vi "HFRR ADV v040.vi"() -> ()   [LabVIEW 2025] (continued)
            w2089 = u32 10000  # timeout (10sec)
            n1729 = VISA Close(VISA resource name=w2084, error in (no error)=w2082) -> (error out=w2085:errorcluster)
            n1730 = local write "Port 1a"(FALSE ("Port 1a")) -> ()
            n1731 = local read "Com Port 1"() -> (w2079:refnum<visa-resource-name>)
            n1732 = call <vilib>:"Clear Errors.vi"("error in (no error)"=w2085) -> ("error out"=w2083:errorcluster)  [unwired: 5 in, 1 out]
            n1733 = call-poly "VISA Configure Serial Port"("VISA resource name"=w2079, "timeout (10sec)"=w2089, "baud rate (9600)"=u32 250000 ("baud rate  2"), "data bits (8)"=u16 8 ("data bits  2"), "parity (0:none)"=w2088, "error in (no error)"=w2083, "stop bits (10: 1 bit)"=w2090, "flow control (0:none)"=w2092) -> ("VISA resource name out"=w2093:refnum<visa-resource-name>, "error out"=w2094:errorcluster)  [unwired: 6 in]
            n1734 = flat-sequence {
              tunnel: w2093 -> [w2096]
              tunnel: w2094 -> [w2095]
              tunnel: [w2096] -> w2086
              tunnel: [w2095] -> w2080
              frame #0 {
                n1735 = Wait (ms)(milliseconds to wait=u32 50) -> ()  [unwired: 1 out]
              }
            }
            "Residual Uno" <- ""
          }
        }
        n1736 = local read "Quit"() -> (w2041:bool)
        "Error Uno" <- w2046
      }
      n1737 = VISA Close(VISA resource name=w2039, error in (no error)=w2038) -> (error out=w2036:errorcluster)
      n1738 = call <vilib>:"Clear Errors.vi"("error in (no error)"=w2036) -> ()  [unwired: 5 in, 2 out]
    }
    frame Enabled {
    }
  }
  n1739 = while {
    stop <- w2107 stop-if-true
    # "V0OLTAGE TO STROKE (peice vise calibration)"
    n1740 = local read "LVDT MIN"() -> (w2099:dbl)
    n1741 = local read "LVDT Peak"() -> (w2098:dbl)
    n1742 = Wait (ms)(milliseconds to wait=u32 10) -> ()  [unwired: 1 out]
    n1743 = formula code="// Dynamic Parameterized Linear Interpolation Node\n// Inputs: vpp_val, voltages (Array), distances (Array)\n// Outputs: stroke\n\nint i = 0;\nint segments = 11; // 12 points make 11 interpolation segments\n\n// 1. Lower Boundary Clamp\nif (vpp_val <= voltages[0]) {\n    stroke = distances[0];\n}\n// 2. Upper Boundary Clamp\nelse if (vpp_val >= voltages[segments]) {\n    stroke = distances[segments];\n}\n// 3. Dynamic Segment Search Loop\nelse {\n    stroke = distances[0]; // Fallback baseline\n    for (i = 0; i < segments; i++) {\n        if (vpp_val >= voltages[i] && vpp_val <= voltages[i+1]) {\n            // Standard linear interpolation formula using array lookups\n            stroke = distances[i] + (vpp_val - voltages[i]) * (distances[i+1] - distances[i]) / (voltages[i+1] - voltages[i]);\n            break; // Segment found, safely exit the loop\n        }\n    }\n}"("vpp_val"=w2098, "voltages"="calibration values", "distances"="STROKE") -> ("stroke"=→"LVDT STROKE":dbl)
    n1744 = local read "Calibration Tare Value"() -> (w2103:dbl)
    n1745 = local read "Calibration Tare"() -> (w2101:bool)
    n1746 = Subtract(x=w2099, y=w2103) -> (x-y=→"LVDT STROKE  Calibration":dbl)
    n1747 = case shown="True" w2101 {
      selector: w2101 -> [_ w2109]
      tunnel: w2099 -> [_ w2110]
      frame False {
      }
      frame True {
        n1748 = Not(x=w2109) -> (.not. x?=w2108:bool)
        n1749 = local write "Calibration Tare"(w2108) -> ()
        "Calibration Tare Value" <- w2110
      }
    }
    n1750 = local read "Quit"() -> (w2107:bool)
  }
  n1751 = while {
    stop <- w2133 stop-if-true
    n1752 = local read "Due read"() -> (w2131:string)
    n1753 = call <vilib>:"High Resolution Polling Wait.vi"("seconds to wait"=0.02) -> ()  [unwired: 10 in, 1 out]
    n1754 = local read "Frictioin Force Raw"() -> (w2113:dbl)
    n1755 = Spreadsheet String To Array(delimiter (Tab)=";", format string="", spreadsheet string=w2131, array type (2D Dbl)=string[] []) -> (array=w2128:string[])
    n1756 = Fract/Exp String To Number(string=w2128) -> (number=w2127:dbl[])  [unwired: 3 in, 1 out]
    n1757 = call <vilib>:"Median Filter PtByPt.vi"("rank"=2, "x"=w2113) -> ("Filtered x"=→"Friction":dbl)  [unwired: 2 in, 1 out]
    n1758 = Index Array(array=w2127) -> (element #1=→"Sample Temperature":dbl, element #2=→"Target Sample Temperature":dbl, element #3=→"Current Duty Cycle":dbl, element #4=→"Ambient Temperature":dbl, element #5=→"Dac Status":dbl, element #6=→"Vpp":dbl, element #7=→"Active Error Code":dbl, element #8=→"Kp":dbl, element #9=→"Ki":dbl, element #10=→"Kd":dbl, element #11=→"SampleRaw":dbl, element #12=→"AmbRaw":dbl)  [unwired: 12 in]
    n1759 = local read "Quit"() -> (w2133:bool)
  }
  n1760 = while {
    shift-right: [w2147] -> w43
    shift-left: _ -> [w2139]
    shift-right: [w2134] -> w42
    shift-left: errorcluster {"status"=FALSE, "code"=0, "source"="Init"} ("error out") -> [w2141]
    tunnel: [w2136] -> w46
    tunnel: [w2146] -> _
    i -> [w2146]
    stop <- w2136 stop-if-true
    n1761 = local read "Com Port 2"() -> (w2140:refnum<visa-resource-name>)
    n1762 = local read "Port 2a"() -> (w2142:bool)
    n1763 = Unbundle(w2141) -> ("status"=→"Port 4":bool)  [unwired: 2 out]
    n1764 = call <vilib>:"High Resolution Polling Wait.vi"("seconds to wait"=0.02) -> ()  [unwired: 10 in, 1 out]
    n1765 = local read "Port 4"() -> (w2143:bool)
    n1766 = Not Equal?(x=w2140, y=w2139) -> (x != y?=w2138:bool)
    n1767 = Or(x=w2143, y=w2142) -> (x .or. y?=w2145:bool)
    n1768 = case shown="False" w2145 {
      frame False {
        w2150 = TRUE ("Visible")
        n1769 = property on="Port 2a" class="Bool (strict)"("Visible"=w2150) -> ()  [unwired: 2 in, 2 out]
        n1770 = property on="Port 4" class="Bool (strict)"("Visible"=w2150) -> ()  [unwired: 2 in, 2 out]
      }
      frame True {
        w2151 = TRUE ("Visible")
        n1771 = property on="Port 2a" class="Bool (strict)"("Visible"=w2151) -> ()  [unwired: 2 in, 2 out]
        n1772 = property on="Port 4" class="Bool (strict)"("Visible"=w2151) -> ()  [unwired: 2 in, 2 out]
      }
    }
    n1773 = case shown="True" w2138 {
      tunnel: [w2148 errorcluster {"status"=TRUE, "code"=0, "source"="Init"} ("error out")] -> w2137
      tunnel: w2141 -> [w2148 _]
      frame False {
      }
      frame True {
      }
    }
    n1774 = case shown="No Error" w2137 {
      selector: w2137 -> [w2164 w2195]
      tunnel: [w2157 w2200] -> w2147
      tunnel: [w2165 w2193] -> w2134
      tunnel: w2139 -> [w2166 w2198]
      frame No Error {
        n1775 = property class="Instr" props=["Serial Settings:Number of Bytes at Serial Port"](reference=w2166, error in=w2164) -> (reference out=w2158:refnum<visa-resource-name>, error out=w2163:errorcluster)  [unwired: 1 out]
        n1776 = while {
          tunnel: [w2174] -> w2159
          tunnel: [w2173] -> w2160
          tunnel: w2163 -> [w2172]
          tunnel: w2158 -> [w2171]
          tunnel: [w2170] -> _
          i -> [w2170]
          stop <- TRUE stop-if-true
          n1777 = property class="Instr" props=["Serial Settings:Number of Bytes at Serial Port"](reference=w2171, error in=w2172) -> (reference out=w2176:refnum<visa-resource-name>, error out=w2175:errorcluster)  [unwired: 1 out]
          n1778 = VISA Read(VISA resource name=w2176, byte count=u32 1000, error in (no error)=w2175) -> (VISA resource name out=w2173:refnum<visa-resource-name>, read buffer=→"Due read":string, error out=w2174:errorcluster)  [unwired: 1 out]
        }
        n1779 = local read "Due Write"() -> (w2156:string)
        n1780 = call <vilib>:"Trim Whitespace.vi"("string"=w2156) -> ("trimmed string"=w2155:string)  [unwired: 1 in]
        n1781 = Not Equal?(x=w2155, y="") -> (x != y?=w2161:bool)
        n1782 = VISA Flush I/O Buffer(VISA resource name=w2160) -> (VISA resource name out=w2153:refnum<visa-resource-name>, error out=→"error out 10":errorcluster)  [unwired: 2 in]
        n1783 = case shown="True" w2161 {
          tunnel: w2153 -> [w2178 w2183]
          tunnel: [w2178 w2187] -> w2157
          tunnel: w2159 -> [w2177 w2182]
          tunnel: [w2177 w2185] -> w2165
          tunnel: w2155 -> [_ w2181]
          tunnel: [_ w2184] -> _
          frame False {
            # "DATA  WRITE LOOP"
          }
          frame True {
            n1784 = Concatenate Strings(w2181, "\r\n") -> (w2180:string)
            n1785 = VISA Write(VISA resource name=w2183, write buffer=w2180, error in (no error)=w2182) -> (VISA resource name out=w2187:refnum<visa-resource-name>, return count=w2184:u32, error out=w2186:errorcluster)
            n1786 = flat-sequence {
              tunnel: w2186 -> [w2189]
              tunnel: [w2189] -> w2185
              frame #0 {
                n1787 = local write "Due Write"("" ("Command")) -> ()
                n1788 = Wait (ms)(milliseconds to wait=u32 5) -> ()  [unwired: 1 out]
              }
            }
          }
        }
        "Port 2a" <- TRUE ("Port 2a")
      }
      frame Error {
        w2206 = u16 0 items=["None", "XON/XOFF", "RTS/CTS", "XON/XOFF & RTS/CTS", "DTR/DSR", "XON/XOFF & DTR/DSR"] ("flow control (0:none)  2")
        w2204 = u16 10 items=["1.0"=10, "1.5"=15, "2.0"=20] ("stop bits 2")
        w2202 = u16 0 items=["None", "Odd", "Even", "Mark", "Space"] ("parity 2")
        w2203 = u32 10000  # timeout (10sec)
        n1789 = VISA Clear(VISA resource name=w2198, error in (no error)=w2195) -> (VISA resource name out=w2197:refnum<visa-resource-name>, error out=w2196:errorcluster)
        n1790 = VISA Close(VISA resource name=w2197, error in (no error)=w2196) -> (error out=w2199:errorcluster)
        n1791 = call <vilib>:"Clear Errors.vi"("error in (no error)"=w2199) -> ()  [unwired: 5 in, 2 out]
        n1792 = local write "Port 2a"(FALSE ("Port 2a")) -> ()
        n1793 = local read "Com Port 2"() -> (w2192:refnum<visa-resource-name>)
        "visa due" <- w2192
        n1794 = call-poly "VISA Configure Serial Port"("VISA resource name"=w2192, "timeout (10sec)"=w2203, "baud rate (9600)"=u32 250000 ("baud rate  2"), "data bits (8)"=u16 8 ("data bits  2"), "parity (0:none)"=w2202, "stop bits (10: 1 bit)"=w2204, "flow control (0:none)"=w2206) -> ("VISA resource name out"=w2207:refnum<visa-resource-name>, "error out"=w2208:errorcluster)  [unwired: 7 in]
        n1795 = flat-sequence {
          tunnel: w2207 -> [w2210]
          tunnel: w2208 -> [w2209]
          tunnel: [w2210] -> w2200
          tunnel: [w2209] -> w2193
          frame #0 {
            n1796 = Wait (ms)(milliseconds to wait=u32 50) -> ()  [unwired: 1 out]
          }
        }
        "Residual Due" <- ""
      }
    }
    "error out 9" <- w2134
    n1797 = local read "Quit"() -> (w2136:bool)
    "Error Due" <- w2141
  }
  n1798 = local write "FRICVALZ"(0.0 ("FRICVALZ")) -> ()
  n1799 = property on="RUN" class="Bool (strict)"("Visible"=TRUE) -> ()  [unwired: 2 in, 2 out]
  n1800 = while {
    tunnel: [w2225] -> _
    tunnel: [w2212] -> w56
    i -> [w2225]
    stop <- w2212 stop-if-true
    n1801 = local read "conststatus"() -> (w2216:dbl)
    n1802 = local read "Main Tab"() -> (w2214:T2)
    n1803 = local read "EDIT"() -> (w2231:bool)
    n1804 = local read "Rate"() -> (w2230:dbl)
    n1805 = case shown="True" w2231 {
      tunnel: [FALSE TRUE] -> _
      frame False {
      }
      frame True {
      }
    }
    n1806 = Equal?(x=w2214, y=T29."About" ("Main Tab")) -> (x = y?=w2223:bool)
    n1807 = Equal?(x=w2216, y=0.0) -> (x = y?=w2217:bool)
    n1808 = Divide(x=1.0, y=w2230) -> (x/y=w2226:dbl)
    "Time 2" <- w2226
    n1809 = case shown="True" w2217 {
      frame False {
      }
      frame True {
        # "C:\\WinDucom\\calibrate WO 2391.dcf"
        n1810 = local write "Lan flag"(22) -> ()
        n1811 = local write "conststatus"(10.0 ("rpm value : 2")) -> ()
        n1812 = String To Path(string="C:\\LAB-IQ\\calibrate WO 2465.dcf") -> (path=w2237:path)
        n1813 = Open/Create/Replace File "Open File"(file path (use dialog)=w2237) -> (refnum out=w2235:refnum<file>)  [unwired: 5 in, 2 out]
        n1814 = for {
          N: 23 -> [_]
          tunnel: w2235 -> [w2246]
          i -> [w2240]
          (unwired) TRUE ("line mode (F)")
          n1815 = Read from Text File "Read File"(file (use dialog)=w2246) -> (text=w2245:string)  [unwired: 3 in, 3 out]
          n1816 = Match Pattern(string=w2245, regular expression="]") -> (after substring=w2243:string)  [unwired: 1 in, 3 out]
          n1817 = String Subset(string=w2245, offset (0)=5, length (rest)=10 ("length (rest)")) -> (substring=w2238:string)
          n1818 = Fract/Exp String To Number(string=w2238) -> (number=w2239:dbl)  [unwired: 3 in, 1 out]
          n1819 = Match Pattern(string=w2243, regular expression="-") -> (before substring=w2241:string)  [unwired: 1 in, 3 out]
          n1820 = case shown="10" w2240 {
            tunnel: w2239 -> [_ _ _ _ _ _ _ _ _ _ w2253 _ _ _ _ _ _ _ _ _ _ _ _ _]
            tunnel: w2241 -> [_ _ _ _ w2249 w2250 w2251 _ _ _ _ _ _ _ _ _ _ _ _ _ w2254 w2255 w2256 _]
            frame 0 {
            }
            frame 1 {
            }
            frame 2 {
            }
            frame 3 {
            }
            frame 4 {
              n1821 = local write "Com Port 1"(w2249) -> ()
            }
            frame 5 {
              n1822 = local write "Com Port 2"(w2250) -> ()
              n1823 = local write "visa due"(w2250) -> ()
            }
            frame 6 {
              n1824 = String To Path(string=w2251) -> (path=w2252:path)
              n1825 = local write "File Path"(w2252) -> ()
              "String" <- w2251
            }
            frame 7 {
            }
            frame 8 {
            }
            frame 9 {
            }
            frame 10 {
              n1826 = local write "Language Selection"(w2253) -> ()
            }
            frame 11 {
            }
            frame 12 {
            }
            frame 13 {
            }
            frame 14 {
            }
            frame 15 {
            }
            frame 16 {
            }
            frame 17 {
            }
            frame 18 {
            }
            frame 21 {
            }
            frame 22 {
              n1827 = local write "Com Port 3"(w2254) -> ()
            }
            frame 20 {
              n1828 = local write "Camera Port :"(w2255) -> ()
            }
            frame 19 {
              n1829 = local write "C3 :"(w2256) -> ()
            }
            frame 23, Default {
            }
          }
        }
      }
    }
    n1830 = Select(t=u32 2500 ("milliseconds to wait"), s=w2223, f=u32 500 ("milliseconds to wait")) -> (s? t:f=w2221:u32)
    n1831 = Multiply(x=w2226, y=w2221) -> (x*y=w2228:dbl)
    n1832 = call "Elapsed Time2"("Time Target (s)"=w2228, "Auto Reset"=TRUE) -> ("Time has Elapsed"=w2218:bool)  [unwired: 10 in, 7 out]
    n1833 = case shown="True" w2218 {
      frame False {
      }
      frame True {
        n1834 = stacked-sequence {
          frame #0 {
            # "DATA PROCESSING"
            # "115 mV/N"
            n1835 = local read "Sample Temperature"() -> (w2259:dbl)
            n1836 = local read "RH Numeric:"() -> (→"Humidity ( %RH )":dbl)
            n1837 = local read "FRICVALZ"() -> (w2276:dbl)
            n1838 = local read "Friction"() -> (w2262:dbl)
            n1839 = call <vilib>:"Mean PtByPt.vi"("x"=w2259, "sample length"=100) -> ("mean"=w2258:dbl)  [unwired: 2 in, 1 out]
            "TEMP 2" <- w2258
            "TEMP 3" <- w2258
            n1840 = Subtract(x=w2262, y=w2276) -> (x-y=w2271:dbl)
            "FF 2" <- w2271
            "FF 4" <- w2271
            n1841 = local read "Ambient Temperature"() -> (→"AIR TEMP":dbl)
            n1842 = local read "TEMP"() -> (w2275:dbl)
            n1843 = local write "FF 3"(w2271) -> ()
            n1844 = Compound Arithmetic op=OR("FRICVALZ 4", "FRICVALZ 3", "FRICVALZ 2") -> (w2267:bool)
            n1845 = case shown="True" w2267 {
              tunnel: w2262 -> [_ w2282]
              frame False {
              }
              frame True {
                w2281 = FALSE ("FRICVALZ")
                n1846 = local write "FRICVALZ 3"(w2281) -> ()
                n1847 = local write "FRICVALZ 2"(w2281) -> ()
                n1848 = local write "FRICVALZ 4"(w2281) -> ()
                "FRICVALZ" <- w2282
              }
            }
            n1849 = Not A Number/Path/Refnum?(number/path/refnum=w2275) -> (NaN/Path/Refnum?=w2274:bool)
            n1850 = Not A Number/Path/Refnum?(number/path/refnum=w2271) -> (NaN/Path/Refnum?=w2273:bool)
            n1851 = Divide(x=w2271, y=1.96) -> (x/y=w2268:dbl)
            n1852 = Compound Arithmetic op=OR(w2274, w2273) -> (w2272:bool)
            n1853 = Not A Number/Path/Refnum?(number/path/refnum=w2268) -> (NaN/Path/Refnum?=w2269:bool)
            n1854 = case shown="True" w2272 {
              frame False {
              }
              frame True {
                n1855 = local write "TEMP"(0.0 ("TEMP")) -> ()
                n1856 = local write "FF 2"(0.0 ("FF 2")) -> ()
                n1857 = local write "reinit"(TRUE ("reinit")) -> ()
              }
            }
            n1858 = local write "TEMP"(w2258) -> ()
            n1859 = Select(t=0.0, s=w2269, f=w2268) -> (s? t:f=w2261:dbl)
            "COF 2" <- w2261
            n1860 = local write "COF 3"(w2261) -> ()
          }
        }
      }
    }
    n1861 = Wait (ms)(milliseconds to wait=u32 50) -> ()  [unwired: 1 out]
    n1862 = local read "Quit"() -> (w2212:bool)
    "Rate" <- 2500.0 ("No of Samples")
  }
  n1863 = while {
    tunnel: [w2302] -> _
    tunnel: [w2285] -> w58
    tunnel: w3 -> [_]
    i -> [w2302]
    stop <- w2285 stop-if-true
    # "C:\\LAB-IQ-NXT\\Scar View.exe"
    n1864 = local read "OK Button 16"() -> (w2292:bool)
    n1865 = local read "Main Tab"() -> (w2286:T2)
    n1866 = local read "service 3"() -> (w2287:bool)
    n1867 = local read "OPEN 6"() -> (w2289:bool)
    n1868 = local read "EDIT 2"() -> (w2291:bool)
    n1869 = flat-sequence {
      frame #0 {
        n1870 = stacked-sequence {
          frame #0 {
            n1871 = local read "EDIT"() -> (w2780:bool)
            n1872 = case shown="False" w2780 {
              tunnel: [u8 2 ("Disabled") u8 0 ("Disabled")] -> _
              frame False {
                w2782 = FALSE
                n1873 = local write "Password"("") -> ()
                n1874 = local write "x = y?"(w2782) -> ()
                n1875 = property on="Password" class="Str"("Visible"=w2782) -> ()  [unwired: 2 in, 2 out]
              }
              frame True {
                n1876 = property on="Password" class="Str"("Visible"=TRUE) -> ()  [unwired: 2 in, 2 out]
              }
            }
            "dipl pwd" <- "@143$\n" ("dipl pwd")
          }
          frame #1 {
          }
          frame #2 {
          }
          frame #3 {
          }
          frame #4 {
            n1877 = String To Byte Array(string="Password") -> (unsigned byte array=w2793:u8[])
            n1878 = Search 1D Array(1D array=w2793, element=u8 10) -> (index of element=w2791:i32)  [unwired: 1 in]
            n1879 = Index Array(array=w2793, index=w2791) -> (element=w2792:u8)
            n1880 = Equal?(x=w2792, y=10) -> (x = y?=w2788:bool)
            n1881 = case shown="True" w2788 {
              frame False {
              }
              frame True {
                # "password"
                # "password"
                n1882 = local read "Password"() -> (w2805:string)
                n1883 = String To Byte Array(string=w2805) -> (unsigned byte array=w2808:u8[])
                n1884 = String To Byte Array(string="@143$\n") -> (unsigned byte array=w2795:u8[])
                n1885 = Array Size(array=w2808) -> (size(s)=w2804:i32)
                n1886 = Array Size(array=w2795) -> (size(s)=w2800:i32)
                n1887 = for {
                  N: w2804 -> [_]
                  tunnel: w2808 -> [w2821]
                  tunnel: [w2819] -> w2809 mode=indexing
                  tunnel: w2804 -> [w2816]
                  i -> [w2817]
                  n1888 = Decrement(x=w2816) -> (x-1=w2815:i32)
                  n1889 = Index Array(array=w2821, index=w2817) -> (element=w2820:u8)
                  n1890 = Equal?(x=w2817, y=w2815) -> (x = y?=w2814:bool)
                  n1891 = Number To Decimal String(number=w2820) -> (decimal integer string=w2818:string)  [unwired: 1 in]
                  n1892 = Select(t="", s=w2814, f="\r") -> (s? t:f=w2811:string)
                  n1893 = Concatenate Strings(w2818, w2811) -> (w2819:string)
                }
                n1894 = for {
                  N: w2800 -> [_]
                  tunnel: w2795 -> [w2832]
                  tunnel: [w2830] -> w2798 mode=indexing
                  tunnel: w2800 -> [w2827]
                  i -> [w2828]
                  n1895 = Decrement(x=w2827) -> (x-1=w2826:i32)
                  n1896 = Index Array(array=w2832, index=w2828) -> (element=w2831:u8)
                  n1897 = Equal?(x=w2828, y=w2826) -> (x = y?=w2825:bool)
                  n1898 = Number To Decimal String(number=w2831) -> (decimal integer string=w2829:string)  [unwired: 1 in]
                  n1899 = Select(t="", s=w2825, f="\r") -> (s? t:f=w2822:string)
                  n1900 = Concatenate Strings(w2829, w2822) -> (w2830:string)
                }
                n1901 = local read "file path"() -> (w2794:path)
                n1902 = call <vilib>:"Read Characters From File.vi"("file path (dialog if empty)"=w2794) -> ("character string"=w2807:string)  [unwired: 5 in, 3 out]
                "string" <- w2807
                n1903 = flat-sequence {
                  tunnel: [w2810] -> _
                  frame #0 {
                    w2810 = ""
                    n1904 = local write "Password"(w2810) -> ()
                  }
                }
                n1905 = Concatenate Strings(w2798) -> (w2799:string)
                n1906 = Concatenate Strings(w2807) -> (w2806:string)
                n1907 = Concatenate Strings(w2809) -> (w2802:string)
                n1908 = Equal?(x=w2802, y=w2806) -> (x = y?=w2797:bool)
                n1909 = Equal?(x=w2802, y=w2799) -> (x = y?=w2803:bool)
                n1910 = Or(x=w2797, y=w2803) -> (x .or. y?=→"x = y?":bool)
              }
            }
          }
        }
        n1911 = local read "x = y?"() -> (w2778:bool)
        n1912 = And(x="EDIT", y=w2778) -> (x .and. y?=w2776:bool)
        n1913 = case shown="True" w2776 {
          tunnel: [u8 2 ("Disabled") u8 0 ("Disabled")] -> w2775
          tunnel: [w2982 TRUE ("Visible")] -> w2774
          frame False {
            w2982 = FALSE ("Visible")
            n1914 = local write "EDIT 2"(w2982) -> ()
          }
          frame True {
          }
        }
        n1915 = case shown="True" "SAVE" {
          frame False {
          }
          frame True {
            n1916 = stacked-sequence {
              seq-local: [w2837 _ _] -> [_ w2978 _]
              frame #0 {
                w2833 = 0.0 ("number")
                w2834 = 0.0 ("number")
                (unwired) i16 5 ("precision (6)")
                # "[CH1]    - FF\n[CH2]   - TEMPERATURE\n[CH3]    - Humidity\n[CH4]    - AIR TEMP\n[CH5]\\- Visa Uno\n[CH6] \\- Visa Due\n[CH7]  \\- file path\n[CH8]   - Displacement Gain\n[CHA]   - Stroke Gain\n[CHB]   - Stroke PID Gain\n[CHC]   -Language Selection\n[CHD]   -Power +\n[CHE]   -Power_\n[CHF]   -Heater\n[CHG]   -Humidity Wet\n[CHH]   -Humidity Dry\n[CHI]   -Integral Time"
                n1917 = local read "Language Selection"() -> (w2880:enum16{"English", "Russian"})
                n1918 = Path To String(path="File Path") -> (string=w2896:string)
                n1919 = Number To Fractional String(number=w2833, width (-)=i16 10 ("precision (6)"), precision (6)=i16 5) -> (F-format string=w2887:string)  [unwired: 1 in]
                n1920 = Number To Fractional String(number=w2880, width (-)=i16 10 ("precision (6)"), precision (6)=i16 5) -> (F-format string=w2876:string)  [unwired: 1 in]
                n1921 = Number To Fractional String(number=w2834, width (-)=i16 10 ("precision (6)"), precision (6)=i16 5) -> (F-format string=w2870:string)  [unwired: 1 in]
                n1922 = Number To Fractional String(number=w2834, width (-)=i16 10 ("precision (6)"), precision (6)=i16 5) -> (F-format string=w2867:string)  [unwired: 1 in]
                n1923 = Number To Fractional String(number=w2834, width (-)=i16 10 ("precision (6)"), precision (6)=i16 5) -> (F-format string=w2862:string)  [unwired: 1 in]
                n1924 = Number To Fractional String(number=w2834, width (-)=i16 10 ("precision (6)"), precision (6)=i16 5) -> (F-format string=w2859:string)  [unwired: 1 in]
                n1925 = Number To Fractional String(number=w2834, width (-)=i16 10 ("precision (6)"), precision (6)=i16 5) -> (F-format string=w2854:string)  [unwired: 1 in]
                n1926 = local read "Com Port 1"() -> (w2836:refnum<visa-resource-name>)
                n1927 = local read "Com Port 2"() -> (w2835:refnum<visa-resource-name>)
                n1928 = Concatenate Strings(w2896, "\\" ("string")) -> (w2895:string)
                n1929 = Number To Fractional String(number=w2833, width (-)=i16 10 ("precision (6)"), precision (6)=i16 5) -> (F-format string=w2928:string)  [unwired: 1 in]
                n1930 = Number To Fractional String(number=w2833, width (-)=i16 10 ("precision (6)"), precision (6)=i16 5) -> (F-format string=w2927:string)  [unwired: 1 in]
                n1931 = Number To Fractional String(number=w2833, width (-)=i16 10 ("precision (6)"), precision (6)=i16 5) -> (F-format string=w2921:string)  [unwired: 1 in]
                n1932 = Number To Fractional String(number=w2833, width (-)=i16 10 ("precision (6)"), precision (6)=i16 5) -> (F-format string=w2915:string)  [unwired: 1 in]
                n1933 = Number To Fractional String(number=w2833, width (-)=i16 10 ("precision (6)"), precision (6)=i16 5) -> (F-format string=w2888:string)  [unwired: 1 in]
                n1934 = Concatenate Strings("[CHA]" ("string"), w2887, "- Stroke Gain" ("string"), "\r") -> (w2881:string)
                n1935 = Concatenate Strings("[CHC]" ("string"), w2876, "-Language Selection" ("string"), "\r") -> (w2873:string)
                n1936 = Concatenate Strings("[CHD]" ("string"), w2870, "-Power +" ("string"), "\r") -> (w2852:string)
                n1937 = Concatenate Strings("[CHG]" ("string"), w2859, "-Humidity Wet" ("string"), "\r") -> (w2849:string)
                n1938 = Concatenate Strings("[CHH]" ("string"), w2854, "-Humidity Dry" ("string"), "\r") -> (w2848:string)
                n1939 = Concatenate Strings("[CH1]" ("string"), w2928, " - FF" ("string"), "\r") -> (w2926:string)
                n1940 = Concatenate Strings("[CH2]" ("string"), w2927, " - TEMPERATURE" ("string"), "\r") -> (w2925:string)
                n1941 = Concatenate Strings("[CH3]" ("string"), w2921, " - Humidity" ("string"), "\r") -> (w2918:string)
                n1942 = Concatenate Strings("[CH4]" ("string"), w2915, " - AIR TEMP" ("string"), "\r") -> (w2911:string)
                n1943 = Concatenate Strings("[CH5]" ("string"), w2836, "- Visa Uno" ("string"), "\r") -> (w2904:string)
                n1944 = Concatenate Strings("[CH6]" ("string"), w2835, "- Visa Due" ("string"), "\r") -> (w2899:string)
                n1945 = Concatenate Strings("[CH7]" ("string"), w2895, "- file path" ("string"), "\r") -> (w2898:string)
                n1946 = Concatenate Strings("[CH8]" ("string"), w2888, "- Displacement Gain" ("string"), "\r") -> (w2891:string)
                n1947 = Concatenate Strings("[CHE]" ("string"), w2867, "-Power_" ("string"), "\r") -> (w2851:string)
                n1948 = Concatenate Strings("[CHF]" ("string"), w2862, "-Heater" ("string"), "\r") -> (w2850:string)
                n1949 = Concatenate Strings(w2926, w2925, w2918, w2911, w2904, w2899, w2898, w2891, w2881, w2873, w2852, w2851, w2850, w2849, w2848) -> (w2837:string)
                "gain" <- w2837
              }
              frame #1 {
                w2939 = 0.0 ("number")
                n1950 = local read "Camera Port :"() -> (w2942:string)
                n1951 = local read "C3 :"() -> (w2950:refnum<visa-resource-name>)
                n1952 = local read "Com Port 3"() -> (w2951:refnum<visa-resource-name>)
                n1953 = Concatenate Strings("[CH8]" ("string"), w2942, "- Visa Camera" ("string"), "\r") -> (w2941:string)
                n1954 = Concatenate Strings("[CH7]" ("string"), w2950, "- Visa Humidity" ("string"), "\r") -> (w2946:string)
                n1955 = Number To Fractional String(number=w2939, width (-)=i16 10 ("precision (6)"), precision (6)=i16 5) -> (F-format string=w2966:string)  [unwired: 1 in]
                n1956 = Concatenate Strings("[CHL]" ("string"), w2951, "- Visa humid" ("string"), "\r") -> (w2954:string)
                n1957 = Number To Fractional String(number=w2939, width (-)=i16 10 ("precision (6)"), precision (6)=i16 5) -> (F-format string=w2973:string)  [unwired: 1 in]
                n1958 = Concatenate Strings("[CHK]" ("string"), w2966, "-TEMP INTERCEPT" ("string"), "\r") -> (w2962:string)
                n1959 = Concatenate Strings("[SNO]" ("string"), "" ("string"), "-" ("string"), "\r") -> (w2959:string)
                n1960 = Concatenate Strings("[CHJ]" ("string"), w2973, "-AIR TEMP INTERCEPT" ("string"), "\r") -> (w2963:string)
                n1961 = String To Path(string="C:\\LAB-IQ\\calibrate WO 2465.dcf") -> (path=w2952:path)
                n1962 = Concatenate Strings(w2978, w2963, w2962, w2959, w2954, w2946, w2941) -> (w2977:string)
                n1963 = call <vilib>:"Write Characters To File.vi"("append to file? (new file:F)"=FALSE, "character string"=w2977, "file path (dialog if empty)"=w2952) -> ()  [unwired: 2 in, 1 out]
              }
              frame #2 {
                n1964 = local write "Lan flag"(0.0 ("Lan flag")) -> ()
                n1965 = local write "conststatus"(0.0 ("rpm value : 2")) -> ()
                n1966 = local write "SAVE"(FALSE ("OK Button 14")) -> ()
              }
            }
          }
        }
        n1967 = property on="EDIT 2" class="Bool (strict)"("Visible"=w2774) -> ()  [unwired: 2 in, 2 out]
        n1968 = property on="SAVE" class="Bool (strict)"("Visible"=w2774) -> ()  [unwired: 2 in, 2 out]
        n1969 = property on="visa due" class="CmbBox"("Disabled"=w2775) -> ()  [unwired: 2 in, 2 out]
        n1970 = property on="File Path" class="Path"("Disabled"=w2775) -> ()  [unwired: 2 in, 2 out]
        n1971 = property on="Language Selection" class="Enum (strict)"("Visible"=w2774) -> ()  [unwired: 2 in, 2 out]
        n1972 = property on="SPEED OUT:" class="DigNum (strict)"("Disabled"=w2775) -> ()  [unwired: 2 in, 2 out]
      }
    }
    n1973 = local read "RUN"() -> (w2301:bool)
    n1974 = local read "RUN"() -> (w2299:bool)
    n1975 = case shown="True" "EDIT 3" {
      frame False {
      }
      frame True {
        n1976 = local write "EDIT 3"(FALSE ("EDIT 3")) -> ()
        n1977 = local write "Main Tab"(T2."About" ("Main Tab")) -> ()
      }
    }
    n1978 = case shown="False" w2301 {
      frame False {
        n1979 = local read "stopT"() -> (w2989:bool)
        n1980 = case shown="True" w2989 {
          frame False {
          }
          frame True {
            n1981 = local write "stopT"(FALSE) -> ()
          }
        }
      }
      frame True {
        "stopT" <- TRUE
      }
    }
    n1982 = case shown="False" w2299 {
      frame False {
      }
      frame True {
      }
    }
    n1983 = case shown="True" w2291 {
      frame False {
        n1984 = property on="Password 2" class="Str"("Visible"=FALSE) -> ()  [unwired: 2 in, 2 out]
        n1985 = local write "Password 2"("" ("Password")) -> ()
      }
      frame True {
        n1986 = property on="Password 2" class="Str"("Visible"=TRUE) -> ()  [unwired: 2 in, 2 out]
        n1987 = Equal?(x="Password 2", y="HFRR1234") -> (x = y?=w2314:bool)
        n1988 = case shown="True" w2314 {
          tunnel: "Password 2" -> [w2317 _]
          frame False {
            n1989 = String Length(string=w2317) -> (length=w2318:i32)
            n1990 = Greater Than 0?(x=w2318) -> (x > 0?=w2316:bool)
            n1991 = case shown="False" w2316 {
              frame False {
                n1992 = property on="Password 2" class="Str"("Caption.Text"="Password (Advance Setting)") -> ()  [unwired: 2 in, 2 out]
              }
              frame True {
                n1993 = property on="Password 2" class="Str"("Caption.Text"="Incorrect Password!") -> ()  [unwired: 2 in, 2 out]
              }
            }
          }
          frame True {
            n1994 = local write "EDIT 2"(FALSE ("EDIT 2")) -> ()
            n1995 = local write "Password 2"("" ("Password")) -> ()
            n1996 = local write "Main Tab"(T2."Advance" ("Main Tab")) -> ()
            n1997 = local write "Main Dashboard Buttons"(T1."Advance" ("Main Dashboard Buttons")) -> ()
          }
        }
      }
    }
    n1998 = case shown="True" "Prog Uno" {
      frame False {
      }
      frame True {
        n1999 = stacked-sequence {
          frame #0 {
            n2000 = Delete(path (use dialog)=path "C:/LAB-IQ-NXT/UNOCOMPILE.bat" ("working directory")) -> ()  [unwired: 4 in, 3 out]
          }
          frame #1 {
            n2001 = local read "Com Port 1"() -> (w2756:refnum<visa-resource-name>)
            n2002 = Concatenate Strings("cmd.exe /c \"mode " ("command line"), w2756, ":1200,n,8,1\"\n" ("command line")) -> (w2761:string)
            n2003 = Concatenate Strings(w2761, "CD\\\nCD WinDucom\navrdude -C avrdude.conf -v -patmega328p -carduino -P" ("command line"), w2756, " -b115200 -D -Uflash:w:UNO_V20.hex:i\n" ("command line"), "\r") -> (w2763:string)
            "STR" <- w2763
            n2004 = call <vilib>:"Write Characters To File.vi"("append to file? (new file:F)"=FALSE, "character string"=w2763, "file path (dialog if empty)"=path "C:/LAB-IQ/UNOCOMPILE.bat" ("working directory")) -> ()  [unwired: 2 in, 1 out]
          }
          frame #2 {
            n2005 = disable-structure shown="Disabled" {
              frame Disabled {
                w2767 = "cmd.exe  /c \"C:\\LAB-IQ-NXT\\UNOCOMPILE.bat\"" ("string")
                n2006 = local write "Prog Uno"(FALSE ("run minimized? (F)")) -> ()
                n2007 = call <vilib>:"System Exec.vi"("expected output size  (4096)"=u32 65535, "run minimized? (F)"=FALSE, "wait until completion? (T)"=TRUE ("run minimized? (F)"), "working directory"=path "C:/LAB-IQ-NXT", "standard input"=w2767, "command line"=w2767) -> ("error out"=w2766:errorcluster, "standard output"=→"String 42":string)  [unwired: 2 in, 2 out]
                "error out 3" <- w2766
                n2008 = flat-sequence {
                  tunnel: w2766 -> [_]
                  frame #0 {
                  }
                }
              }
              frame Enabled {
              }
            }
          }
        }
      }
    }
    n2009 = case shown="\"ISO 12156\"" "TEST STANDARD" {
      frame "ASTM D6079", Default {
        w2736 = 50.0 ("Hz")
        w2737 = 53.0 ("Set Rh")
        w2739 = 1.0 ("Set Strk")
        w2738 = 60.0 ("Set Temp")
        # "astm hide"
        n2010 = local write "NORMAL LOAD"(200.0 ("NORMAL LOAD")) -> ()
        n2011 = local write "Set Strk"(w2739) -> ()
        n2012 = local write "Set Hz"(w2736) -> ()
        n2013 = local write "Set Temp"(w2738) -> ()
        n2014 = local write "Set Rh"(w2737) -> ()
        n2015 = local write "test time"(75.0 ("test time")) -> ()
        n2016 = local write "Set Stroke:"(w2739) -> ()
        n2017 = local write "Set Humidity:"(w2737) -> ()
        n2018 = local write "Set Frequency:"(w2736) -> ()
        n2019 = local write "Set Temperature:"(w2738) -> ()
        "Test Standard" <- "ASTM D6079" ("Test Standard 2")
      }
      frame "ISO 12156" {
        n2020 = local write "Set Strk"(1.0 ("Set Strk")) -> ()
        n2021 = local write "NORMAL LOAD"(200.0 ("NORMAL LOAD")) -> ()
        n2022 = local write "Set Temp"(60.0 ("Set Temp")) -> ()
        n2023 = local write "test time"(75.0 ("test time")) -> ()
        n2024 = local write "Set Hz"(50.0 ("Hz")) -> ()
        n2025 = local write "Set Rh"(53.0 ("Set Rh")) -> ()
      }
      frame "CEC F-096-A-06" {
        n2026 = local write "Set Strk"(1.0 ("Set Strk")) -> ()
        n2027 = local write "NORMAL LOAD"(200.0 ("NORMAL LOAD")) -> ()
        n2028 = local write "Set Temp"(60.0 ("Set Temp")) -> ()
        n2029 = local write "test time"(75.0 ("test time")) -> ()
        n2030 = local write "Set Hz"(50.0 ("Hz")) -> ()
        n2031 = local write "Set Rh"(53.0 ("Set Rh")) -> ()
      }
      frame "Custom" {
      }
    }
    n2032 = Or(x=w2289, y=w2287) -> (x .or. y?=w2288:bool)
    n2033 = case shown="\"About\"" w2286 {
      tunnel: [T29."Acquire" ("Main Tab") T29."Compare Files" ("Main Tab") T29."About" ("Main Tab")] -> w2297
      frame "Acquire", Default {
      }
      frame "Compare Files" {
      }
      frame "About" {
      }
    }
    n2034 = Or(x=w2292, y="OPEN") -> (x .or. y?=w2293:bool)
    n2035 = case shown="True" w2293 {
      tunnel: w2292 -> [_ w2325]
      frame False {
      }
      frame True {
        n2036 = stacked-sequence {
          tunnel: w2325 -> [_ w2392 _ _]
          frame #0 {
            w2341 = "  " ("String 6")
            n2037 = local write "OPEN"(FALSE ("open")) -> ()
            n2038 = local read "string1 2"() -> (w2329:string)
            n2039 = local read "string1 3"() -> (w2328:string)
            n2040 = local read "string1 4"() -> (w2327:string)
            n2041 = property on="OPEN" class="Bool (strict)"("Visible"=FALSE) -> ()  [unwired: 2 in, 2 out]
            n2042 = local write "String 6"(w2341) -> ()
            n2043 = local write "String 7"(w2341) -> ()
            n2044 = local write "String 8"(w2341) -> ()
            n2045 = local write "String 12"(w2341) -> ()
            n2046 = local read "OK Button 16"() -> (w2326:bool)
            n2047 = String To Path(string=w2329) -> (path=w2337:path)
            n2048 = String To Path(string=w2328) -> (path=w2336:path)
            n2049 = String To Path(string=w2327) -> (path=w2335:path)
            n2050 = case shown="True" w2326 {
              tunnel: [w2342 w2343] -> w2330
              frame False {
                n2051 = local read "string1"() -> (w2342:string)
              }
              frame True {
                n2052 = local read "String Indicator 4"() -> (w2343:string)
              }
            }
            n2053 = Open/Create/Replace File "Open File"(file path (use dialog)=w2337) -> (refnum out=w2333:refnum<file>)  [unwired: 5 in, 2 out]
            n2054 = Open/Create/Replace File "Open File"(file path (use dialog)=w2336) -> (refnum out=w2332:refnum<file>)  [unwired: 5 in, 2 out]
            n2055 = Open/Create/Replace File "Open File"(file path (use dialog)=w2335) -> (refnum out=w2331:refnum<file>)  [unwired: 5 in, 2 out]
            n2056 = while {
              tunnel: w2333 -> [w2355]
              i -> [w2351]
              stop <- w2350 continue-if-true
              (unwired) TRUE ("line mode (F)")
              n2057 = Read from Text File "Read File"(file (use dialog)=w2355) -> (text=w2352:string)  [unwired: 3 in, 3 out]
              n2058 = local write "Numeric 11"(w2351) -> ()
              n2059 = String Length(string=w2352) -> (length=w2354:i32)
              n2060 = Greater?(x=w2354, y=1) -> (0:w2350:bool)
            }
            n2061 = while {
              tunnel: w2332 -> [w2361]
              i -> [w2357]
              stop <- w2356 continue-if-true
              (unwired) TRUE ("line mode (F)")
              n2062 = Read from Text File "Read File"(file (use dialog)=w2361) -> (text=w2358:string)  [unwired: 3 in, 3 out]
              n2063 = local write "Numeric 12"(w2357) -> ()
              n2064 = String Length(string=w2358) -> (length=w2360:i32)
              n2065 = Greater?(x=w2360, y=1) -> (0:w2356:bool)
            }
            n2066 = while {
              tunnel: w2331 -> [w2367]
              i -> [w2363]
              stop <- w2362 continue-if-true
              (unwired) TRUE ("line mode (F)")
              n2067 = Read from Text File "Read File"(file (use dialog)=w2367) -> (text=w2364:string)  [unwired: 3 in, 3 out]
              n2068 = local write "Numeric 13"(w2363) -> ()
              n2069 = String Length(string=w2364) -> (length=w2366:i32)
              n2070 = Greater?(x=w2366, y=1) -> (0:w2362:bool)
            }
            n2071 = String To Path(string=w2330) -> (path=w2338:path)
            n2072 = Open/Create/Replace File "Open File"(file path (use dialog)=w2338) -> (refnum out=w2334:refnum<file>)  [unwired: 5 in, 2 out]
            n2073 = while {
              tunnel: w2334 -> [w2349]
              i -> [w2345]
              stop <- w2344 continue-if-true
              (unwired) TRUE ("line mode (F)")
              n2074 = Read from Text File "Read File"(file (use dialog)=w2349) -> (text=w2346:string)  [unwired: 3 in, 3 out]
              n2075 = local write "Numeric 8"(w2345) -> ()
              n2076 = String Length(string=w2346) -> (length=w2348:i32)
              n2077 = Greater?(x=w2348, y=1) -> (0:w2344:bool)
            }
          }
          frame #1 {
            w2519 = FALSE ("ACTUAL   MERGE")
            # "Sample Temp"
            # "ECR"
            # "COF"
            # "Time\nCOF\nFF\nTemp"
            n2078 = case shown="True" w2392 {
              tunnel: [w2539 w2540] -> w2393
              frame False {
                n2079 = local read "string1"() -> (w2539:string)
              }
              frame True {
                n2080 = local read "String Indicator 4"() -> (w2540:string)
              }
            }
            n2081 = local read "string1 3"() -> (w2437:string)
            n2082 = String To Path(string=w2393) -> (path=w2524:path)
            n2083 = String To Path(string=w2437) -> (path=w2535:path)
            n2084 = local read "Numeric 12"() -> (w2521:i32)
            n2085 = local read "Numeric 8"() -> (w2523:i32)
            n2086 = local read "string1 2"() -> (w2438:string)
            n2087 = local read "string1 4"() -> (w2436:string)
            n2088 = Open/Create/Replace File "Open File"(file path (use dialog)=w2524) -> (refnum out=w2538:refnum<file>, error out=w2537:errorcluster)  [unwired: 5 in, 1 out]
            n2089 = Open/Create/Replace File "Open File"(file path (use dialog)=w2535) -> (refnum out=w2531:refnum<file>, error out=w2532:errorcluster)  [unwired: 5 in, 1 out]
            n2090 = for {
              N: w2523 -> [_]
              tunnel: w2538 -> [w2686]
              tunnel: w2537 -> [w2685]
              tunnel: [w2675] -> w2450 mode=indexing
              tunnel: [w2673] -> w2507 mode=indexing
              tunnel: [w2674] -> w2502 mode=indexing
              tunnel: w2519 -> [_]
              tunnel: [w2667] -> w2504 mode=indexing
              tunnel: [w2663] -> w2473 mode=indexing
              tunnel: [w2659] -> w2448 mode=indexing
              tunnel: [w2655] -> w2429 mode=indexing
              tunnel: [w2650] -> w2389 mode=indexing
              (unwired) TRUE ("line mode (F)")
              # "freq"
              # "Stroke"
              # "Time"
              # "CoF"
              # "Humidity"
              # "Temp"
              # "Air Temp"
              # "ECR"
              n2091 = Read from Text File "Read File"(file (use dialog)=w2686, error in=w2685) -> (text=w2651:string)  [unwired: 2 in, 3 out]
              n2092 = local write "String 6"(w2651) -> ()
              n2093 = String Subset(string=w2651, offset (0)=0, length (rest)=14 ("length (rest)")) -> (substring=w2679:string)
              n2094 = String Subset(string=w2651, offset (0)=35, length (rest)=9 ("length (rest)")) -> (substring=w2676:string)
              n2095 = String Subset(string=w2651, offset (0)=15, length (rest)=9 ("length (rest)")) -> (substring=w2682:string)
              n2096 = Fract/Exp String To Number(string=w2679) -> (number=w2675:dbl)  [unwired: 3 in, 1 out]
              n2097 = Fract/Exp String To Number(string=w2676) -> (number=w2674:dbl)  [unwired: 3 in, 1 out]
              n2098 = Fract/Exp String To Number(string=w2682) -> (number=w2673:dbl)  [unwired: 3 in, 1 out]
              n2099 = String Subset(string=w2651, offset (0)=85, length (rest)=9 ("length (rest)")) -> (substring=w2652:string)
              n2100 = String Subset(string=w2651, offset (0)=25, length (rest)=9 ("length (rest)")) -> (substring=w2658:string)
              n2101 = String Subset(string=w2651, offset (0)=55, length (rest)=9 ("length (rest)")) -> (substring=w2660:string)
              n2102 = String Subset(string=w2651, offset (0)=45, length (rest)=9 ("length (rest)")) -> (substring=w2666:string)
              n2103 = String Subset(string=w2651, offset (0)=65, length (rest)=9 ("length (rest)")) -> (substring=w2672:string)
              n2104 = Fract/Exp String To Number(string=w2658) -> (number=w2655:dbl)  [unwired: 3 in, 1 out]
              n2105 = Fract/Exp String To Number(string=w2652) -> (number=w2650:dbl)  [unwired: 3 in, 1 out]
              n2106 = Fract/Exp String To Number(string=w2660) -> (number=w2659:dbl)  [unwired: 3 in, 1 out]
              n2107 = Fract/Exp String To Number(string=w2666) -> (number=w2663:dbl)  [unwired: 3 in, 1 out]
              n2108 = Fract/Exp String To Number(string=w2672) -> (number=w2669:dbl)  [unwired: 3 in, 1 out]
              n2109 = Add(x=w2669, y=0.0) -> (x+y=w2667:dbl)
            }
            n2110 = for {
              N: w2521 -> [_]
              tunnel: w2532 -> [w2612]
              tunnel: w2531 -> [w2611]
              tunnel: [w2601] -> w2490 mode=indexing
              tunnel: [w2599] -> w2488 mode=indexing
              tunnel: [w2600] -> w2484 mode=indexing
              tunnel: w2519 -> [_]
              tunnel: [w2593] -> w2486 mode=indexing
              tunnel: [w2589] -> w2468 mode=indexing
              tunnel: [w2585] -> w2444 mode=indexing
              tunnel: [w2582] -> w2425 mode=indexing
              tunnel: [w2578] -> w2384 mode=indexing
              (unwired) 9 ("length (rest)")
              (unwired) 9 ("length (rest)")
              (unwired) TRUE ("line mode (F)")
              n2111 = Read from Text File "Read File"(file (use dialog)=w2611, error in=w2612) -> (text=w2579:string)  [unwired: 2 in, 3 out]
              n2112 = local write "String 8"(w2579) -> ()
              n2113 = String Subset(string=w2579, offset (0)=85) -> (substring=w2581:string)  [unwired: 1 in]
              n2114 = String Subset(string=w2579, offset (0)=35, length (rest)=9 ("length (rest)")) -> (substring=w2602:string)
              n2115 = String Subset(string=w2579, offset (0)=55, length (rest)=9 ("length (rest)")) -> (substring=w2587:string)
              n2116 = String Subset(string=w2579, offset (0)=25) -> (substring=w2583:string)  [unwired: 1 in]
              n2117 = String Subset(string=w2579, offset (0)=15, length (rest)=9 ("length (rest)")) -> (substring=w2608:string)
              n2118 = String Subset(string=w2579, offset (0)=0, length (rest)=14 ("length (rest)")) -> (substring=w2605:string)
              n2119 = String Subset(string=w2579, offset (0)=45, length (rest)=9 ("length (rest)")) -> (substring=w2592:string)
              n2120 = String Subset(string=w2579, offset (0)=65, length (rest)=9 ("length (rest)")) -> (substring=w2598:string)
              n2121 = Fract/Exp String To Number(string=w2581) -> (number=w2578:dbl)  [unwired: 3 in, 1 out]
              n2122 = Fract/Exp String To Number(string=w2602) -> (number=w2600:dbl)  [unwired: 3 in, 1 out]
              n2123 = Fract/Exp String To Number(string=w2587) -> (number=w2585:dbl)  [unwired: 3 in, 1 out]
              n2124 = Fract/Exp String To Number(string=w2583) -> (number=w2582:dbl)  [unwired: 3 in, 1 out]
              n2125 = Fract/Exp String To Number(string=w2608) -> (number=w2599:dbl)  [unwired: 3 in, 1 out]
              n2126 = Fract/Exp String To Number(string=w2605) -> (number=w2601:dbl)  [unwired: 3 in, 1 out]
              n2127 = Fract/Exp String To Number(string=w2592) -> (number=w2589:dbl)  [unwired: 3 in, 1 out]
              n2128 = Fract/Exp String To Number(string=w2598) -> (number=w2595:dbl)  [unwired: 3 in, 1 out]
              n2129 = Add(x=w2595, y=0.0) -> (x+y=w2593:dbl)
            }
            n2130 = String To Path(string=w2438) -> (path=w2536:path)
            n2131 = String To Path(string=w2436) -> (path=w2530:path)
            n2132 = local read "Numeric 11"() -> (w2520:i32)
            n2133 = local read "Numeric 13"() -> (w2522:i32)
            n2134 = Open/Create/Replace File "Open File"(file path (use dialog)=w2536) -> (refnum out=w2534:refnum<file>, error out=w2533:errorcluster)  [unwired: 5 in, 1 out]
            n2135 = Open/Create/Replace File "Open File"(file path (use dialog)=w2530) -> (refnum out=w2529:refnum<file>, error out=w2528:errorcluster)  [unwired: 5 in, 1 out]
            n2136 = for {
              N: w2520 -> [_]
              tunnel: w2534 -> [w2649]
              tunnel: w2533 -> [w2648]
              tunnel: [w2638] -> w2500 mode=indexing
              tunnel: [w2636] -> w2498 mode=indexing
              tunnel: [w2637] -> w2493 mode=indexing
              tunnel: w2519 -> [_]
              tunnel: [w2630] -> w2495 mode=indexing
              tunnel: [w2626] -> w2471 mode=indexing
              tunnel: [w2622] -> w2446 mode=indexing
              tunnel: [w2618] -> w2427 mode=indexing
              tunnel: [w2613] -> w2385 mode=indexing
              (unwired) TRUE ("line mode (F)")
              n2137 = Read from Text File "Read File"(file (use dialog)=w2649, error in=w2648) -> (text=w2614:string)  [unwired: 2 in, 3 out]
              n2138 = local write "String 7"(w2614) -> ()
              n2139 = String Subset(string=w2614, offset (0)=85, length (rest)=9 ("length (rest)")) -> (substring=w2617:string)
              n2140 = String Subset(string=w2614, offset (0)=35, length (rest)=9 ("length (rest)")) -> (substring=w2639:string)
              n2141 = String Subset(string=w2614, offset (0)=55, length (rest)=9 ("length (rest)")) -> (substring=w2625:string)
              n2142 = String Subset(string=w2614, offset (0)=25, length (rest)=9 ("length (rest)")) -> (substring=w2619:string)
              n2143 = String Subset(string=w2614, offset (0)=45, length (rest)=9 ("length (rest)")) -> (substring=w2627:string)
              n2144 = String Subset(string=w2614, offset (0)=0, length (rest)=14 ("length (rest)")) -> (substring=w2642:string)
              n2145 = String Subset(string=w2614, offset (0)=15, length (rest)=9 ("length (rest)")) -> (substring=w2645:string)
              n2146 = String Subset(string=w2614, offset (0)=65, length (rest)=9 ("length (rest)")) -> (substring=w2631:string)
              n2147 = Fract/Exp String To Number(string=w2617) -> (number=w2613:dbl)  [unwired: 3 in, 1 out]
              n2148 = Fract/Exp String To Number(string=w2639) -> (number=w2637:dbl)  [unwired: 3 in, 1 out]
              n2149 = Fract/Exp String To Number(string=w2625) -> (number=w2622:dbl)  [unwired: 3 in, 1 out]
              n2150 = Fract/Exp String To Number(string=w2619) -> (number=w2618:dbl)  [unwired: 3 in, 1 out]
              n2151 = Fract/Exp String To Number(string=w2627) -> (number=w2626:dbl)  [unwired: 3 in, 1 out]
              n2152 = Fract/Exp String To Number(string=w2642) -> (number=w2638:dbl)  [unwired: 3 in, 1 out]
              n2153 = Fract/Exp String To Number(string=w2645) -> (number=w2636:dbl)  [unwired: 3 in, 1 out]
              n2154 = Fract/Exp String To Number(string=w2631) -> (number=w2634:dbl)  [unwired: 3 in, 1 out]
              n2155 = Add(x=w2634, y=0.0) -> (x+y=w2630:dbl)
            }
            n2156 = for {
              N: w2522 -> [_]
              tunnel: w2529 -> [w2577]
              tunnel: w2528 -> [w2576]
              tunnel: [w2566] -> w2482 mode=indexing
              tunnel: [w2565] -> w2475 mode=indexing
              tunnel: w2519 -> [_]
              tunnel: [w2554] -> w2480 mode=indexing
              tunnel: [w2559] -> w2477 mode=indexing
              tunnel: [w2555] -> w2467 mode=indexing
              tunnel: [w2550] -> w2442 mode=indexing
              tunnel: [w2546] -> w2423 mode=indexing
              tunnel: [w2541] -> w2383 mode=indexing
              (unwired) 1.0 ("x")
              (unwired) TRUE ("line mode (F)")
              n2157 = Read from Text File "Read File"(file (use dialog)=w2577, error in=w2576) -> (text=w2542:string)  [unwired: 2 in, 3 out]
              n2158 = local write "String 12"(w2542) -> ()
              n2159 = String Subset(string=w2542, offset (0)=85, length (rest)=9 ("length (rest)")) -> (substring=w2544:string)
              n2160 = String Subset(string=w2542, offset (0)=35, length (rest)=9 ("length (rest)")) -> (substring=w2567:string)
              n2161 = String Subset(string=w2542, offset (0)=55, length (rest)=9 ("length (rest)")) -> (substring=w2552:string)
              n2162 = String Subset(string=w2542, offset (0)=25, length (rest)=9 ("length (rest)")) -> (substring=w2548:string)
              n2163 = String Subset(string=w2542, offset (0)=45, length (rest)=9 ("length (rest)")) -> (substring=w2557:string)
              n2164 = String Subset(string=w2542, offset (0)=15, length (rest)=9 ("length (rest)")) -> (substring=w2573:string)
              n2165 = String Subset(string=w2542, offset (0)=0, length (rest)=14 ("length (rest)")) -> (substring=w2570:string)
              n2166 = String Subset(string=w2542, offset (0)=65, length (rest)=9 ("length (rest)")) -> (substring=w2560:string)
              n2167 = Fract/Exp String To Number(string=w2544) -> (number=w2541:dbl)  [unwired: 3 in, 1 out]
              n2168 = Fract/Exp String To Number(string=w2567) -> (number=w2565:dbl)  [unwired: 3 in, 1 out]
              n2169 = Fract/Exp String To Number(string=w2552) -> (number=w2550:dbl)  [unwired: 3 in, 1 out]
              n2170 = Fract/Exp String To Number(string=w2548) -> (number=w2546:dbl)  [unwired: 3 in, 1 out]
              n2171 = Fract/Exp String To Number(string=w2557) -> (number=w2555:dbl)  [unwired: 3 in, 1 out]
              n2172 = Fract/Exp String To Number(string=w2573) -> (number=w2554:dbl)  [unwired: 3 in, 1 out]
              n2173 = Fract/Exp String To Number(string=w2570) -> (number=w2566:dbl)  [unwired: 3 in, 1 out]
              n2174 = Fract/Exp String To Number(string=w2560) -> (number=w2563:dbl)  [unwired: 3 in, 1 out]
              n2175 = Add(x=w2563, y=0.0) -> (x+y=w2559:dbl)
            }
            n2176 = Delete From Array(array=w2425, index=0) -> (array with subset deleted=w2398:dbl[])  [unwired: 1 in, 1 out]
            n2177 = Delete From Array(array=w2488, index=0) -> (array with subset deleted=w2461:dbl[])  [unwired: 1 in, 1 out]
            n2178 = Delete From Array(array=w2468, index=0) -> (array with subset deleted=w2456:dbl[])  [unwired: 1 in, 1 out]
            n2179 = Delete From Array(array=w2486, index=0) -> (array with subset deleted=w2487:dbl[])  [unwired: 1 in, 1 out]
            n2180 = call-poly <vilib>:"Mean.vi"("X"=w2398) -> ("mean"=→"КОФ2 4":dbl)  [unwired: 1 out]
            n2181 = call-poly <vilib>:"Mean.vi"("X"=w2461) -> ("mean"=→"КОФ3":dbl)  [unwired: 1 out]
            n2182 = call-poly <vilib>:"Mean.vi"("X"=w2456) -> ("mean"=→"CP3":dbl)  [unwired: 1 out]
            n2183 = Delete From Array(array=w2450, index=0) -> (array with subset deleted=w2377:dbl[])  [unwired: 1 in, 1 out]
            n2184 = Delete From Array(array=w2389, index=0) -> (array with subset deleted=w2376:dbl[])  [unwired: 1 in, 1 out]
            n2185 = Delete From Array(array=w2429, index=0) -> (array with subset deleted=w2400:dbl[])  [unwired: 1 in, 1 out]
            n2186 = Delete From Array(array=w2507, index=0) -> (array with subset deleted=w2462:dbl[])  [unwired: 1 in, 1 out]
            n2187 = Delete From Array(array=w2473, index=0) -> (array with subset deleted=w2458:dbl[])  [unwired: 1 in, 1 out]
            "array w/ subset deleted" <- w2458
            n2188 = Delete From Array(array=w2504, index=0) -> (array with subset deleted=w2505:dbl[])  [unwired: 1 in, 1 out]
            n2189 = call-poly <vilib>:"Mean.vi"("X"=w2400) -> ("mean"=→"КОФ2 2":dbl)  [unwired: 1 out]
            n2190 = call-poly <vilib>:"Mean.vi"("X"=w2462) -> ("mean"=→"КОФ1":dbl)  [unwired: 1 out]
            n2191 = Bundle "Bundle"(w2377, w2376) -> (w2382:cluster{dbl[], dbl[]})  [unwired: 1 in]
            n2192 = Bundle "Bundle"(w2377, w2505) -> (w2369:cluster{dbl[], dbl[]})  [unwired: 1 in]
            n2193 = Delete From Array(array=w2384, index=0) -> (array with subset deleted=w2372:dbl[])  [unwired: 1 in, 1 out]
            n2194 = Delete From Array(array=w2385, index=0) -> (array with subset deleted=w2374:dbl[])  [unwired: 1 in, 1 out]
            n2195 = Delete From Array(array=w2495, index=0) -> (array with subset deleted=w2496:dbl[])  [unwired: 1 in, 1 out]
            n2196 = Delete From Array(array=w2383, index=0) -> (array with subset deleted=w2370:dbl[])  [unwired: 1 in, 1 out]
            n2197 = Delete From Array(array=w2477, index=0) -> (array with subset deleted=w2478:dbl[])  [unwired: 1 in, 1 out]